vi "UHR-Fleezers Control (host) - 12.0(oscillate_test).vi"() -> ()   [LabVIEW 2014] (continued)
        n1224 = Divide(x=w1672, y="APD Integration Time (s)") -> (x/y=w1675:dbl)
        n1225 = Multiply(x=2.0, y=w1675) -> (x*y=w1674:dbl)
        n1226 = local write "APD Samples/FIFO Acq."(w1675) -> ()
        n1227 = local write "APD Elements/DMA read"(w1674) -> ()
      }
      event "Number of F/B Scans (AOD)", "Scan Speed (nm/s)", "Scan BD", "Initial D (MHz)", "Step Size (nm)", "Scan Range (nm)", "Wiggle amp 1 (units?)": Value Change {
        w1743 = 123.0  # AOM cal (nm/MHz)
        n1228 = event-data() -> ()  [unwired: 7 out]
        n1229 = local read "BD 1 Frequency 1 (MHz)"() -> (w1726:dbl)
        n1230 = local read "AOM X Cal (nm/MHz)"() -> (w1718:dbl)
        n1231 = local read "BD 2 Frequency 1 (MHz)"() -> (w1732:dbl)
        n1232 = local read "X RF Frequency Limits (MHz)"() -> (w1730:T17)
        n1233 = local read "Y RF Frequency Limits (MHz)"() -> (w1727:T17)
        n1234 = Negate(x="Scan Range (nm)") -> (-x=w1696:dbl)
        n1235 = Divide(x=w1696, y=w1718) -> (x/y=w1700:dbl)
        n1236 = Select(t=w1730, s="Scan BD", f=w1727) -> (s? t:f=w1729:T17)
        n1237 = Select(t=w1726, s="Scan BD", f=w1732) -> (s? t:f=w1731:dbl)
        n1238 = Unbundle By Name(w1729) -> ("Maximum"=w1738:dbl, "Minimum"=w1737:dbl)
        n1239 = Add(x=w1700, y=w1731) -> (x+y=w1735:dbl)
        n1240 = Divide(x=w1696, y="Step Size (nm)") -> (x/y=w1715:dbl)
        n1241 = Divide(x="Step Size (nm)", y=w1718) -> (x/y=w1724:dbl)
        n1242 = Absolute Value(x=w1715) -> (abs(x)=w1699:dbl)
        n1243 = Sign(1:w1696) -> (0:w1697:dbl)
        n1244 = In Range and Coerce(upper limit=w1738, x=w1735, lower limit=w1737) -> (coerced(x)=w1734:dbl, In Range?=w1736:bool)
        n1245 = To Unsigned Quad Integer(1:w1699) -> (0:w1714:u64)
        "Scan steps (AOD)" <- w1714
        n1246 = call "IR AOM freq to word.vi"("Frequency In (MHz)"=w1724) -> ("Frequency Word Out (double)"=w1721:dbl)
        n1247 = Multiply(x=w1697, y=w1721) -> (x*y=w1698:dbl)
        n1248 = Subtract(x=w1735, y=w1734) -> (x-y=w1733:dbl)
        n1249 = To Quad Integer(1:w1698) -> (0:w1720:i64)
        "Incr. int (AOD)" <- w1720
        n1250 = Subtract(x=w1700, y=w1733) -> (x-y=w1719:dbl)
        "Scan Range (MHz)" <- w1719
        n1251 = Select(t=w1700, s=w1736, f=w1719) -> (s? t:f=w1739:dbl)
        n1252 = Multiply(x=w1719, y=w1718) -> (x*y=w1717:dbl)
        n1253 = Decrement(x=w1714) -> (x-1=w1767:u64)
        n1254 = Negate(x=w1717) -> (-x=w1713:dbl)
        n1255 = local write "Scan Range (nm)"(w1713) -> ()
        n1256 = Divide(x=w1739, y=w1767) -> (x/y=w1723:dbl)
        "Scan Increment (MHz)" <- w1723
        n1257 = call "IR AOM freq to word.vi"("Frequency In (MHz)"=w1723) -> ("Frequency Word Out (double)"=w1722:dbl)
        n1258 = Divide(x="Step Size (nm)", y="Scan Speed (nm/s)") -> (x/y=w1710:dbl)
        n1259 = To Quad Integer(1:w1722) -> ()  [unwired: 1 out]
        n1260 = local read "Number Interlace Sets"() -> (w1694:u8)
        n1261 = local read "AI Count (ticks)"() -> (w1695:u32)
        n1262 = local read "Total Counts (ticks)"() -> (w1693:u32)
        n1263 = local read "# Samples/trap"() -> (w1725:u32)
        n1264 = Multiply(x=w1695, y=w1694) -> (x*y=w1692:u32)
        n1265 = Divide(x=w1693, y=w1692) -> (x/y=w1691:dbl)
        n1266 = Select(t=w1726, s="Scan BD", f=w1732) -> (s? t:f=w1764:dbl)
        "Initial freq. (MHz)" <- w1764
        n1267 = Add(x=w1739, y=w1764) -> (x+y=→"Final freq. (MHz)":dbl)
        n1268 = Divide(x=w1693, y=40000000.0) -> (x/y=w1709:dbl)
        n1269 = Divide(x=w1710, y=w1709) -> (x/y=w1708:dbl)
        n1270 = To Unsigned Quad Integer(1:w1708) -> (0:w1683:u64)
        n1271 = Quotient & Remainder(x=w1683, y=u64 2) -> (x-y*floor(x/y)=w1687:u64)  [unwired: 1 out]
        n1272 = Equal?(x=w1687, y=u64 0) -> (x = y?=w1685:bool)
        n1273 = Decrement(x=w1683) -> (x-1=w1684:u64)
        n1274 = Select(t=w1683, s=w1685, f=w1684) -> (s? t:f=w1682:u64)
        "Cycles/step (AOD)" <- w1682
        n1275 = xnode "Read/Write Control"("FPGA VI Reference In"=w1775, "error in"=w1774, "Scan steps"=w1714, "Number of scans"="Number of F/B Scans (AOD)", "Cycles per step"=w1682, "Scan freq.  increment"=w1720, "Scan BD"="Scan BD") -> ("error out"=w1773:errorcluster)  [unwired: 1 out]
        n1276 = Multiply(x=w1714, y=w1682) -> (x*y=w1768:u64)
        n1277 = Multiply(x=w1768, y=u64 2) -> (x*y=w1690:u64)
        n1278 = Multiply(x=w1691, y=w1690) -> (x*y=w1689:dbl)
        "Data points/scan (f/b)" <- w1689
        n1279 = Multiply(x=w1689, y="Number of F/B Scans (AOD)") -> (x*y=w1771:dbl)
        "Data points/scans" <- w1771
        n1280 = Divide(x=w1771, y=w1725) -> (x/y=→"N sets should be saved":dbl)
        n1281 = Multiply(x=w1768, y=w1709) -> (x*y=w1707:dbl)
        "Time/Scan (s) (AOD)" <- w1707
        n1282 = Select(t=w1739, s="Scan BD", f=0.0) -> (s? t:f=w1765:dbl)
        n1283 = Select(t=0.0, s="Scan BD", f=w1739) -> (s? t:f=w1761:dbl)
        n1284 = local read "BD 2 Frequency 2 (MHz)"() -> (w1757:dbl)
        n1285 = local read "BD 1 Frequency 2 (MHz)"() -> (w1760:dbl)
        n1286 = Add(x=w1761, y=w1732) -> (x+y=w1758:dbl)
        n1287 = Add(x=w1726, y=w1765) -> (x+y=w1759:dbl)
        n1288 = Multiply(x=w1707, y=2.0) -> (x*y=w1706:dbl)
        n1289 = Multiply(x=w1706, y="Number of F/B Scans (AOD)") -> (x*y=w1703:dbl)
        n1290 = Divide(x=w1703, y=60.0) -> (x/y=→"Time to Finish All (min)":dbl)
        n1291 = Add(x="Trap 2 Bead Size (nm)", y="Trap 1 Bead Size (nm)") -> (x+y=w1747:dbl)
        n1292 = Divide(x=w1747, y=2.0) -> (x/y=w1741:dbl)
        n1293 = Subtract(x=w1758, y=w1757) -> (x-y=w1755:dbl)
        n1294 = Subtract(x=w1759, y=w1760) -> (x-y=w1756:dbl)
        n1295 = local read "Initial D (MHz)"() -> (w1744:dbl)
        n1296 = Square(x=w1755) -> (x^2=w1754:dbl)
        n1297 = Square(x=w1756) -> (x^2=w1753:dbl)
        n1298 = Add(x=w1753, y=w1754) -> (x+y=w1752:dbl)
        n1299 = Square Root(x=w1752) -> (sqrt(x)=w1751:dbl)
        "Final D (MHz)" <- w1751
        n1300 = Multiply(x=w1743, y=w1751) -> (x*y=w1750:dbl)
        n1301 = Multiply(x=w1744, y=w1743) -> (x*y=w1742:dbl)
        n1302 = Subtract(x=w1742, y=w1741) -> (x-y=→"Initial sep (nm)":dbl)
        n1303 = Subtract(x=w1750, y=w1741) -> (x-y=→"Final sep (nm)":dbl)
      }
      event "Freq or Amp switch first", "Swap F1 and F2", "Freq switch delay", "Amp switch delay": Value Change {
        n1304 = event-data() -> ()  [unwired: 7 out]
        n1305 = local read "Freq or Amp switch first"() -> (w1776:bool)
        n1306 = local read "Amp switch delay"() -> (w1777:u16)
        n1307 = local read "Freq switch delay"() -> (w1779:u16)
        n1308 = local read "Swap F1 and F2"() -> (w1778:bool)
        n1309 = xnode "Read/Write Control"("FPGA VI Reference In"=w1782, "error in"=w1781, "Freq switch delay"=w1779, "Swap F1 and F2"=w1778, "Amp switch delay"=w1777, "Freq or Amp switch first"=w1776) -> ("error out"=w1780:errorcluster)  [unwired: 1 out]
      }
      event "Scan steps (MCL)", "Number of scans (MCL)", "Scan Range (V)\n(of steps)", "2D or 1D Scan", "N APD Samp/step", "Fast Scan Dir", "Continuous MCL Scanning", "Scan lines (y)": Value Change {
        w1784 = 32767.0 ("y")
        n1310 = event-data() -> ()  [unwired: 7 out]
        n1311 = Select(t="Scan lines (y)", s="2D or 1D Scan", f="Number of scans (MCL)") -> (s? t:f=w1789:u64)
        n1312 = Decrement(x="Scan steps (MCL)") -> (x-1=w1805:u64)
        n1313 = Divide(x="Scan Range (V)\n(of steps)", y=w1805) -> (x/y=w1804:dbl)
        "Desired Scan Incr (V)" <- w1804
        n1314 = local read "APD Integration Time (s)"() -> (w1797:dbl)
        n1315 = Multiply(x=w1804, y=w1784) -> (x*y=w1813:dbl)
        n1316 = Divide(x=w1813, y=10.0) -> (x/y=w1803:dbl)
        "Desired incr (int)" <- w1803
        n1317 = local read "Update Count (MCL)"() -> (w1809:u32)
        n1318 = Round Toward -Infinity(1:w1803) -> (0:w1812:dbl)
        n1319 = To Word Integer(number=w1812) -> (16bit integer=w1787:i16)
        "Actual Incr. int (MCL)" <- w1787
        n1320 = Multiply(x=w1797, y=40000000.0) -> (x*y=w1810:dbl)
        n1321 = Divide(x=w1810, y=w1809) -> (x/y=w1808:dbl)
        n1322 = Multiply(x=i16 10, y=w1787) -> (x*y=w1785:i16)
        n1323 = Multiply(x="N APD Samp/step", y=w1808) -> (x*y=w1807:dbl)
        "Cycles/step (MCL)" <- w1807
        n1324 = Divide(x=w1785, y=w1784) -> (x/y=→"Actual MCL Inc (V)":dbl)
        n1325 = Multiply(x="N APD Samp/step", y="Scan steps (MCL)") -> (x*y=w1799:dbl)
        n1326 = local read "APD Samples/FIFO Acq."() -> (w1796:dbl)
        n1327 = Multiply(x=w1799, y=u64 2) -> (x*y=w1798:dbl)
        "Data points/scan (f+b)" <- w1798
        n1328 = Multiply(x=w1798, y=w1789) -> (x*y=w1816:dbl)
        "Data points/scans (MCL)" <- w1816
        n1329 = Multiply(x=w1797, y=w1798) -> (x*y=w1790:dbl)
        "Time/f+b scan (s) (MCL)" <- w1790
        n1330 = Divide(x=w1816, y=w1796) -> (x/y=→"N sets should be saved (MCL)":dbl)
        n1331 = Multiply(x=w1790, y=w1789) -> (x*y=→"Total Time (s)":dbl)
        n1332 = Not(x="Fast Scan Dir") -> (.not. x?=w1794:bool)
        n1333 = xnode "Read/Write Control"("FPGA VI Reference In"=w1820, "error in"=w1819, "Scan steps (MCL)"="Scan steps (MCL)", "Number of scans (MCL)"=w1789, "Cycles per step (MCL)"=w1807, "Scan freq.  increment (MCL)"=w1787, "1D or 2D Scan?"="2D or 1D Scan", "MCL Scan Axis"=w1794, "Cont. Scan (MCL)"="Continuous MCL Scanning") -> ("error out"=w1818:errorcluster)  [unwired: 1 out]
      }
      event "Read Cal": Value Change {
        w1822 = 1000.0 ("y")
        n1334 = event-data() -> ()  [unwired: 7 out]
        n1335 = local read "Save file name"() -> (w1847:path)
        n1336 = local write "Read Cal"(FALSE ("Read Cal")) -> ()
        n1337 = Strip Path(path=w1847) -> (stripped path=w1846:path)  [unwired: 1 out]
        n1338 = Path To String(path=w1846) -> (string=w1845:string)
        n1339 = Concatenate Strings(w1845, "\\current.cal" ("string")) -> (w1843:string)
        n1340 = String To Path(string=w1843) -> (path=w1842:path)
        n1341 = Open/Create/Replace File(file path (use dialog)=w1842, operation (0:open)=T30."open", access (0:read/write)=enum16{"read/write", "read-only", "write-only"}."read-only") -> (refnum out=w1850:refnum<file>, error out=w1836:errorcluster)  [unwired: 1 in, 3 out]
        n1342 = Deny Access(4:w1836, 7:w1850) -> (0:w1835:errorcluster, 3:w1841:refnum<file>)  [unwired: 1 out]
        n1343 = Read from Binary File(5:0.0, 8:w1835, 9:T29."big-endian, network order" ("byte order (0:big-endian, network order)"), 10:-1 ("count (1)"), 11:w1841) -> (0:w1834:errorcluster, 2:w1832:dbl[], 3:w1837:refnum<file>)  [unwired: 2 out]
        n1344 = Array To Cluster(array=w1832) -> (cluster=w1831:T32)
        n1345 = Unbundle(w1831) -> ("[0]"=w1830:dbl, "[1]"=w1829:dbl, "[2]"=w1828:dbl, "[3]"=w1827:dbl, "[4]"=w1826:dbl, "[5]"=w1825:dbl)
        n1346 = Close File(refnum=w1837, error in=w1834) -> (error out=→"Read cal error":errorcluster)  [unwired: 1 out]
        n1347 = Multiply(x=w1825, y=w1822) -> (x*y=w1823:dbl)
        n1348 = local write "T2 k_x (pN/nm)"(w1827) -> ()
        n1349 = local write "T1 k_x (pN/nm)"(w1828) -> ()
        n1350 = local write "T1 a_x (nm/V)"(w1830) -> ()
        n1351 = local write "T2 a_x (nm/V)"(w1829) -> ()
        n1352 = Multiply(x=w1826, y=w1822) -> (x*y=w1824:dbl)
        n1353 = local write "T1 offset_x (mV)"(w1824) -> ()
        n1354 = local write "T2 offset_x (mV)"(w1823) -> ()
      }
      event "Read FX file": Value Change {
        n1355 = event-data() -> ()  [unwired: 7 out]
        n1356 = local write "Read FX file"(FALSE ("Read residual")) -> ()
        n1357 = local read "Save file name"() -> (w1875:path)
        n1358 = Strip Path(path=w1875) -> (stripped path=w1874:path)  [unwired: 1 out]
        n1359 = Path To String(path=w1874) -> (string=w1873:string)
        n1360 = Concatenate Strings(w1873, "\\current.cal" ("string")) -> (w1871:string)
        n1361 = String To Path(string=w1871) -> (path=w1870:path)
        n1362 = Open/Create/Replace File(file path (use dialog)=w1870, operation (0:open)=T30."open", access (0:read/write)=enum16{"read/write", "read-only", "write-only"}."read-only") -> (refnum out=w1867:refnum<file>, error out=w1864:errorcluster)  [unwired: 3 in, 1 out]
        n1363 = Deny Access(4:w1864, 7:w1867) -> (0:w1863:errorcluster, 3:w1866:refnum<file>)  [unwired: 1 in]
        n1364 = Read from Binary File(5:0.0, 8:w1863, 9:T29."big-endian, network order" ("byte order (0:big-endian, network order)"), 10:-1 ("count"), 11:w1866) -> (0:w1859:errorcluster, 2:w1853:dbl[], 3:w1860:refnum<file>)  [unwired: 1 in, 1 out]
        n1365 = Index Array(array=w1853, index=6) -> (element=→"Bad fit error":dbl)
        n1366 = Index Array(array=w1853, index=7) -> (element=→"Fit offset":dbl)
        n1367 = Index Array(array=w1853, index=8) -> (element=→"Hyst. error":dbl)
        n1368 = Close File(refnum=w1860, error in=w1859) -> ()  [unwired: 2 out]
      }
      event "Abort MCL Scan": Value Change {
        n1369 = event-data() -> ()  [unwired: 7 out]
        n1370 = local write "MCL Scanning"(FALSE ("MCL Scanning")) -> ()
        n1371 = xnode "Read/Write Control"("FPGA VI Reference In"=w1880, "error in"=w1879, "Abort scan (MCL)"="Abort MCL Scan") -> ("error out"=w1878:errorcluster)  [unwired: 1 out]
      }
      event "Update Count (MCL)": Value Change {
        n1372 = event-data() -> ()  [unwired: 7 out]
        n1373 = xnode "Read/Write Control"("FPGA VI Reference In"=w1884, "error in"=w1883, "MCL count"="Update Count (MCL)") -> ("error out"=w1882:errorcluster)  [unwired: 1 out]
      }
      event "Phase adjust (MCL)", "+ phase (MCL)", "- phase (MCL)": Value Change {
        n1374 = event-data() -> ()  [unwired: 7 out]
        n1375 = Negate(x="Phase adjust (MCL)") -> (-x=w1893:i16)
        n1376 = Select(t=w1893, s="- phase (MCL)", f="Phase adjust (MCL)") -> (s? t:f=w1891:i16)
        n1377 = Or(x="- phase (MCL)", y="+ phase (MCL)") -> (x .or. y?=w1886:bool)
        n1378 = xnode "Read/Write Control"("FPGA VI Reference In"=w1895, "error in"=w1894, "Phase count adjustment (MCL)"=w1891) -> ("FPGA VI Reference Out"=w1887:T22, "error out"=w1888:errorcluster)
        n1379 = xnode "Read/Write Control"("FPGA VI Reference In"=w1887, "error in"=w1888, "+ phase (MCL)"=w1886) -> ("error out"=w1885:errorcluster)  [unwired: 1 out]
      }
      event "Abort AOD Scan": Value Change {
        n1380 = event-data() -> ()  [unwired: 7 out]
        n1381 = xnode "Read/Write Control"("FPGA VI Reference In"=w1899, "error in"=w1898, "Abort scan"="Abort AOD Scan") -> ("error out"=w1897:errorcluster)  [unwired: 1 out]
      }
      event "Continuous AOD Scanning": Value Change {
        n1382 = event-data() -> ()  [unwired: 7 out]
        n1383 = xnode "Read/Write Control"("FPGA VI Reference In"=w1903, "error in"=w1902, "Cont. Scan"="Continuous AOD Scanning") -> ("error out"=w1901:errorcluster)  [unwired: 1 out]
      }
      event "Index": Value Change {
        n1384 = event-data() -> ()  [unwired: 7 out]
        n1385 = call "Create new save file.vi"("Insert"="", "Ext"=".dat" ("string"), "Index In"="Index") -> ("Path Out"=→"Save file name":path, "Index Out"=w1904:dbl)
        "Save index" <- w1904
        n1386 = local write "Index"(w1904) -> ()
      }
      event "AO1", "AO2": Value Change {
        w1919 = 10.0 ("y")
        w1918 = 32767.0 ("y")
        n1387 = event-data() -> ()  [unwired: 7 out]
        n1388 = local read "AO2"() -> (w1917:dbl)
        n1389 = local read "AO1"() -> (w1914:dbl)
        n1390 = Multiply(x=w1914, y=w1918) -> (x*y=w1913:dbl)
        n1391 = Multiply(x=w1917, y=w1918) -> (x*y=w1916:dbl)
        n1392 = Divide(x=w1913, y=w1919) -> (x/y=w1912:dbl)
        n1393 = Divide(x=w1916, y=w1919) -> (x/y=w1915:dbl)
        n1394 = To Word Integer(number=w1912) -> (16bit integer=w1920:i16)
        n1395 = To Word Integer(number=w1915) -> (16bit integer=w1921:i16)
        n1396 = xnode "Read/Write Control"("FPGA VI Reference In"=w1911, "error in"=w1910, "AO1"=w1920, "AO2"=w1921) -> ("error out"=w1909:errorcluster)  [unwired: 1 out]
      }
      event "Inject Pump 1": Value Change {
        n1397 = event-data() -> ()  [unwired: 7 out]
        n1398 = local read "Use Harvard pumps\nfor beads (else Chemyx)"() -> (w1923:bool)
        n1399 = case shown="True" w1923 {
          tunnel: "Inject Pump 1" -> [w1927 w1965]
          tunnel: w1922 -> [_ w1966]
          frame False {
            n1400 = local read "Pump write delay (ms)"() -> (w1926:dbl)
            n1401 = local read "Chemyx Syringe Pump Serial Port"() -> (w1925:refnum<visa-resource-name>)
            n1402 = case shown="True" w1927 {
              tunnel: w1926 -> [w1933 w1947]
              tunnel: w1925 -> [w1930 w1946]
              frame False {
                n1403 = flat-sequence {
                  tunnel: w1930 -> [w1934]
                  tunnel: [w1934] -> w1931
                  tunnel: w1933 -> [_]
                  tunnel: [w1937] -> w1932
                  tunnel: w1931 -> [w1937]
                  tunnel: w1932 -> [w1938]
                  tunnel: [w1938] -> w1928
                  tunnel: [w1940] -> w1929
                  tunnel: w1928 -> [w1940]
                  tunnel: w1929 -> [w1942]
                  frame #0 {
                    n1404 = call "Write to pump.vi"("string"="enter pump1", "VISA resource name"=w1934) -> ()  [unwired: 1 out]
                  }
                  frame #1 {
                    n1405 = Wait (ms)(milliseconds to wait="Pump pause delay (ms)") -> ()  [unwired: 1 out]
                  }
                  frame #2 {
                    n1406 = call "Write to pump.vi"("string"="stop", "VISA resource name"=w1938) -> ()  [unwired: 1 out]
                  }
                  frame #3 {
                    n1407 = Wait (ms)(milliseconds to wait=u32 500) -> ()  [unwired: 1 out]
                  }
                  frame #4 {
                    n1408 = call "Write to pump.vi"("string"="stop", "VISA resource name"=w1942) -> ()  [unwired: 1 out]
                  }
                }
              }
              frame True {
                n1409 = flat-sequence {
                  tunnel: w1946 -> [w1956]
                  tunnel: w1947 -> [w1951]
                  tunnel: w1947 -> [w1958]
                  tunnel: w1946 -> [w1959]
                  tunnel: [w1959] -> w1944
                  tunnel: [w1961] -> w1945
                  tunnel: w1944 -> [w1961]
                  tunnel: w1945 -> [w1963]
                  frame #0 {
                    n1410 = local read "All Pump Parameters"() -> (w1950:T5)
                    n1411 = Unbundle By Name(w1950) -> ("Pump 1"=w1957:T33)
                    n1412 = call "Set pump parameters.vi"("Pump write delay (ms)"=w1951, "Volume (uL)"="Ch 1 Inject Volume (uL)", "Rate (uL/h)"="Ch 1 Inject Rate (ul/h)", "Units"=4.0, "Pump #"=1.0, "Pump Parameters In"=w1957, "VISA resource name"=w1956) -> ("Pump Parameters Out"=w1949:T33)  [unwired: 3 in]
                    n1413 = Bundle By Name(cluster=w1950, "Pump 1"=w1949) -> (w1948:T5)
                    n1414 = local write "All Pump Parameters"(w1948) -> ()
                  }
                  frame #1 {
                    n1415 = Wait (ms)(milliseconds to wait=w1958) -> ()  [unwired: 1 out]
                  }
                  frame #2 {
                    n1416 = call "Write to pump.vi"("string"="start", "VISA resource name"=w1959) -> ()  [unwired: 1 out]
                  }
                  frame #3 {
                    n1417 = Wait (ms)(milliseconds to wait=u32 500) -> ()  [unwired: 1 out]
                  }
                  frame #4 {
                    n1418 = call "Write to pump.vi"("string"="start", "VISA resource name"=w1963) -> ()  [unwired: 1 out]
                  }
                }
              }
            }
          }
          frame True {
            n1419 = case shown="True" w1965 {
              tunnel: w1966 -> [w1967 w1977]
              frame False {
                n1420 = flat-sequence {
                  tunnel: w1967 -> [w1969]
                  frame #0 {
                    n1421 = local write "Flushing P1"(FALSE ("Flushing P1")) -> ()
                    n1422 = Concatenate Strings("stop" ("string"), "\r") -> (w1971:string)
                    n1423 = VISA Write(VISA resource name=w1969, write buffer=w1971) -> ()  [unwired: 1 in, 3 out]
                  }
                  frame #1 {
                    n1424 = property on="Clear Volume P1" class="Bool (strict)"("Val(Sgnl)"=TRUE ("Value (Signaling)")) -> ()  [unwired: 2 in, 2 out]
                  }
                }
              }
              frame True {
                n1425 = local read "Normal Flow Rate (ul/h) P1"() -> (w1975:dbl)
                n1426 = Number To Decimal String(number=w1975) -> (decimal integer string=w1981:string)  [unwired: 1 in]
                n1427 = Concatenate Strings("irate  " ("string"), w1981, " u/h" ("string"), "\r") -> (w1979:string)
                n1428 = VISA Write(VISA resource name=w1977, write buffer=w1979) -> (VISA resource name out=w1976:refnum<visa-resource-name>)  [unwired: 1 in, 2 out]
                n1429 = Concatenate Strings("irun" ("string"), "\r") -> (w1983:string)
                n1430 = VISA Write(VISA resource name=w1976, write buffer=w1983) -> ()  [unwired: 1 in, 3 out]
              }
            }
          }
        }
      }
      event "Inject Pump 3": Value Change {
        n1431 = event-data() -> ()  [unwired: 7 out]
        n1432 = local read "Use Harvard pumps\nfor beads (else Chemyx)"() -> (w1986:bool)
        n1433 = case shown="True" w1986 {
          tunnel: "Inject Pump 3" -> [w1990 w2029]
          tunnel: w1985 -> [_ w2028]
          frame False {
            n1434 = local read "Pump write delay (ms)"() -> (w1989:dbl)
            n1435 = case shown="True" w1990 {
              tunnel: w1989 -> [w1996 w2010]
              tunnel: "Chemyx Syringe Pump Serial Port" -> [w1993 w2009]
              frame False {
                n1436 = flat-sequence {
                  tunnel: w1993 -> [w1997]
                  tunnel: [w1997] -> w1994
                  tunnel: w1996 -> [_]
                  tunnel: [w2000] -> w1995
                  tunnel: w1994 -> [w2000]
                  tunnel: w1995 -> [w2001]
                  tunnel: [w2001] -> w1991
                  tunnel: [w2003] -> w1992
                  tunnel: w1991 -> [w2003]
                  tunnel: w1992 -> [w2005]
                  frame #0 {
                    n1437 = call "Write to pump.vi"("string"="enter pump3", "VISA resource name"=w1997) -> ()  [unwired: 1 out]
                  }
                  frame #1 {
                    n1438 = local read "Pump pause delay (ms)"() -> (w1999:u32)
                    n1439 = Wait (ms)(milliseconds to wait=w1999) -> ()  [unwired: 1 out]
                  }
                  frame #2 {
                    n1440 = call "Write to pump.vi"("string"="stop", "VISA resource name"=w2001) -> ()  [unwired: 1 out]
                  }
                  frame #3 {
                    n1441 = Wait (ms)(milliseconds to wait=u32 0) -> ()  [unwired: 1 out]
                  }
                  frame #4 {
                    n1442 = call "Write to pump.vi"("string"="stop", "VISA resource name"=w2005) -> ()  [unwired: 1 out]
                  }
                }
              }
              frame True {
                n1443 = flat-sequence {
                  tunnel: w2009 -> [w2019]
                  tunnel: w2010 -> [w2014]
                  tunnel: w2010 -> [w2021]
                  tunnel: w2009 -> [w2022]
                  tunnel: [w2022] -> w2008
                  tunnel: [w2025] -> w2007
                  tunnel: w2008 -> [w2025]
                  tunnel: w2007 -> [w2026]
                  frame #0 {
                    n1444 = local read "All Pump Parameters"() -> (w2013:T5)
                    n1445 = Unbundle By Name(w2013) -> ("Pump 3"=w2020:T33)
                    n1446 = call "Set pump parameters.vi"("Pump write delay (ms)"=w2014, "Volume (uL)"="Ch 3 Inject Volume (uL)", "Rate (uL/h)"="Ch 3 Inject Rate (ul/h)", "Units"=4.0, "Pump #"=3.0, "Pump Parameters In"=w2020, "VISA resource name"=w2019) -> ("Pump Parameters Out"=w2012:T33)  [unwired: 3 in]
                    n1447 = Bundle By Name(cluster=w2013, "Pump 3"=w2012) -> (w2011:T5)
                    n1448 = local write "All Pump Parameters"(w2011) -> ()
                  }
                  frame #1 {
                    n1449 = Wait (ms)(milliseconds to wait=w2021) -> ()  [unwired: 1 out]
                  }
                  frame #2 {
                    n1450 = call "Write to pump.vi"("string"="start", "VISA resource name"=w2022) -> ()  [unwired: 1 out]
                  }
                  frame #3 {
                    n1451 = Wait (ms)(milliseconds to wait=u32 500) -> ()  [unwired: 1 out]
                  }
                  frame #4 {
                    n1452 = call "Write to pump.vi"("string"="start", "VISA resource name"=w2026) -> ()  [unwired: 1 out]
                  }
                }
              }
            }
          }
          frame True {
            n1453 = case shown="True" w2029 {
              tunnel: w2028 -> [w2030 w2037]
              frame False {
                n1454 = flat-sequence {
                  tunnel: w2030 -> [w2032]
                  frame #0 {
                    n1455 = local write "Flushing P3"(FALSE ("Flushing P3")) -> ()
                    n1456 = Concatenate Strings("stop" ("string"), "\r") -> (w2034:string)
                    n1457 = VISA Write(VISA resource name=w2032, write buffer=w2034) -> ()  [unwired: 1 in, 3 out]
                  }
                  frame #1 {
                    n1458 = property on="Clear Volume P3" class="Bool (strict)"("Val(Sgnl)"=TRUE ("Value (Signaling)")) -> ()  [unwired: 2 in, 2 out]
                  }
                }
              }
              frame True {
                n1459 = local read "Normal Flow Rate (ul/h) P3"() -> (w2038:dbl)
                n1460 = Number To Decimal String(number=w2038) -> (decimal integer string=w2044:string)  [unwired: 1 in]
                n1461 = Concatenate Strings("irate  " ("string"), w2044, " u/h" ("string"), "\r") -> (w2042:string)
                n1462 = VISA Write(VISA resource name=w2037, write buffer=w2042) -> (VISA resource name out=w2040:refnum<visa-resource-name>)  [unwired: 1 in, 2 out]
                n1463 = Concatenate Strings("irun" ("string"), "\r") -> (w2046:string)
                n1464 = VISA Write(VISA resource name=w2040, write buffer=w2046) -> ()  [unwired: 1 in, 3 out]
              }
            }
          }
        }
      }
      event "Inject Pump 2": Value Change {
        n1465 = event-data() -> ()  [unwired: 7 out]
        n1466 = local read "Pump write delay (ms)"() -> (w2050:dbl)
        n1467 = local read "Chemyx Syringe Pump Serial Port"() -> (w2048:refnum<visa-resource-name>)
        n1468 = flat-sequence {
          tunnel: w2048 -> [w2063]
          tunnel: w2050 -> [w2059]
          tunnel: "Inject Pump 2" -> [_]
          tunnel: w2050 -> [w2065]
          tunnel: w2048 -> [w2066]
          frame #0 {
            n1469 = local read "All Pump Parameters"() -> (w2058:T5)
            n1470 = Multiply(x=60.0, y="Flush Center Ch Rate (ul/m)") -> (x*y=w2055:dbl)
            n1471 = Unbundle By Name(w2058) -> ("Pump 2"=w2064:T33)
            n1472 = call "Set pump parameters.vi"("Pump write delay (ms)"=w2059, "Volume (uL)"="Flush Center Ch Volume (uL)", "Rate (uL/h)"=w2055, "Units"=3.0, "Pump #"=2.0, "Pump Parameters In"=w2064, "VISA resource name"=w2063) -> ("Pump Parameters Out"=w2057:T33)  [unwired: 3 in]
            n1473 = Bundle By Name(cluster=w2058, "Pump 2"=w2057) -> (w2056:T5)
            n1474 = Add(x="Flush Center Ch Volume (uL)", y="Total Volume\nFlushed (uL)") -> (x+y=w2052:dbl)
            n1475 = local write "All Pump Parameters"(w2056) -> ()
            n1476 = local write "Total Volume\nFlushed (uL)"(w2052) -> ()
          }
          frame #1 {
            n1477 = Wait (ms)(milliseconds to wait=w2065) -> ()  [unwired: 1 out]
          }
          frame #2 {
            n1478 = call "Write to pump.vi"("string"="start", "VISA resource name"=w2066) -> ()  [unwired: 1 out]
          }
        }
      }
      event "Sample Channel\nFlow": Value Change {
        n1479 = event-data() -> ()  [unwired: 7 out]
        n1480 = case shown="True" "Sample Channel\nFlow" {
          tunnel: w2069 -> [w2070 w2076]
          frame False {
            n1481 = flat-sequence {
              tunnel: w2070 -> [w2072]
              frame #0 {
                n1482 = local write "Flushing samp"(FALSE ("Flushing samp")) -> ()
                n1483 = Concatenate Strings("stop" ("string"), "\r") -> (w2075:string)
                n1484 = VISA Write(VISA resource name=w2072, write buffer=w2075) -> ()  [unwired: 1 in, 3 out]
              }
            }
          }
          frame True {
            n1485 = local read "Normal Flow rate (mL/h)"() -> (w2086:dbl)
            n1486 = Number To Decimal String(number=w2086) -> (decimal integer string=w2085:string)  [unwired: 1 in]
            n1487 = Concatenate Strings("irate " ("string"), w2085, " u/h" ("string"), "\r") -> (w2081:string)
            n1488 = VISA Write(VISA resource name=w2076, write buffer=w2081) -> (VISA resource name out=w2080:refnum<visa-resource-name>)  [unwired: 1 in, 2 out]
            n1489 = Concatenate Strings("irun" ("string"), "\r") -> (w2077:string)
            n1490 = VISA Write(VISA resource name=w2080, write buffer=w2077) -> ()  [unwired: 1 in, 3 out]
          }
        }
      }
      event "Start Flow": Value Change {
        n1491 = event-data() -> ()  [unwired: 7 out]
        n1492 = local write "Sample Channel\nFlow"(TRUE ("Sample Channel\nFlow")) -> ()
        n1493 = local write "Start Flow"(FALSE ("Start Flow")) -> ()
        n1494 = Concatenate Strings("irun" ("string"), "\r") -> (w2091:string)
        n1495 = VISA Write(VISA resource name=w2087, write buffer=w2091) -> ()  [unwired: 1 in, 3 out]
      }
      event "Stop Flow": Value Change {
        w2093 = FALSE ("Stop Flow")
        n1496 = event-data() -> ()  [unwired: 7 out]
        n1497 = local write "Stop Flow"(w2093) -> ()
        n1498 = local write "Sample Channel\nFlow"(w2093) -> ()
        n1499 = Concatenate Strings("stop" ("string"), "\r") -> (w2096:string)
        n1500 = VISA Write(VISA resource name=w2094, write buffer=w2096) -> ()  [unwired: 1 in, 3 out]
      }
      event "Normal Flow rate (mL/h)": Value Change {
        n1501 = event-data() -> ()  [unwired: 7 out]
        n1502 = Number To Decimal String(number="Normal Flow rate (mL/h)") -> (decimal integer string=w2103:string)  [unwired: 1 in]
        n1503 = Concatenate Strings("irate  " ("string"), w2103, " u/h" ("string"), "\r") -> (w2102:string)
        n1504 = VISA Write(VISA resource name=w2099, write buffer=w2102) -> ()  [unwired: 1 in, 3 out]
      }
      event "Flush Sample": Value Change {
        n1505 = event-data() -> ()  [unwired: 7 out]
        n1506 = flat-sequence {
          tunnel: w2105 -> [w2133]
          frame #0 {
            # "set parameters (rate, volume) for flush, clear volume"
            n1507 = Number To Decimal String(number="Flush rate (mL/m)") -> (decimal integer string=w2129:string)  [unwired: 1 in]
            n1508 = local write "Sample Channel\nFlow"(TRUE ("Sample Channel\nFlow")) -> ()
            n1509 = Concatenate Strings("irate  " ("string"), w2129, " u/m" ("string"), "\r") -> (w2131:string)
            n1510 = VISA Write(VISA resource name=w2133, write buffer=w2131) -> (VISA resource name out=w2127:refnum<visa-resource-name>)  [unwired: 1 in, 2 out]
            n1511 = Number To Decimal String(number="Flush volume (mL)") -> (decimal integer string=w2118:string)  [unwired: 1 in]
            n1512 = Reciprocal(x="Flush rate (mL/m)") -> (1/x=w2112:dbl)
            n1513 = Concatenate Strings("tvolume  " ("string"), w2118, " u" ("string"), "\r") -> (w2116:string)
            n1514 = Multiply(x=w2112, y="Flush volume (mL)") -> (x*y=w2110:dbl)
            n1515 = VISA Write(VISA resource name=w2127, write buffer=w2116) -> (VISA resource name out=w2115:refnum<visa-resource-name>)  [unwired: 1 in, 2 out]
            n1516 = Multiply(x=w2110, y=60.0) -> (x*y=→"Samp Flush Time (s)":dbl)
            n1517 = Concatenate Strings("cvolume" ("string"), "\r") -> (w2114:string)
            n1518 = VISA Write(VISA resource name=w2115, write buffer=w2114) -> (VISA resource name out=w2125:refnum<visa-resource-name>)  [unwired: 1 in, 2 out]
            n1519 = Concatenate Strings("irun" ("string"), "\r") -> (w2123:string)
            n1520 = VISA Write(VISA resource name=w2125, write buffer=w2123) -> ()  [unwired: 1 in, 3 out]
          }
          frame #1 {
            "Flushing samp" <- TRUE ("Boolean")
          }
        }
      }
      event "Flush Pump 3": Value Change {
        n1521 = event-data() -> ()  [unwired: 7 out]
        n1522 = flat-sequence {
          tunnel: w2135 -> [w2138]
          frame #0 {
            # "set paramaters (rate, volume) for flush, clear volume"
            n1523 = Number To Decimal String(number="Flush rate (uL/m) P3") -> (decimal integer string=w2160:string)  [unwired: 1 in]
            n1524 = local write "Inject Pump 3"(TRUE ("Inject Pump 3")) -> ()
            n1525 = Concatenate Strings("irate  " ("string"), w2160, " u/m" ("string"), "\r") -> (w2162:string)
            n1526 = VISA Write(VISA resource name=w2138, write buffer=w2162) -> (VISA resource name out=w2158:refnum<visa-resource-name>)  [unwired: 1 in, 2 out]
            n1527 = Reciprocal(x="Flush rate (uL/m) P3") -> (1/x=w2142:dbl)
            n1528 = Number To Decimal String(number="Volume (uL) P3") -> (decimal integer string=w2149:string)  [unwired: 1 in]
            n1529 = Multiply(x="Volume (uL) P3", y=w2142) -> (x*y=w2141:dbl)
            n1530 = Concatenate Strings("tvolume  " ("string"), w2149, " u" ("string"), "\r") -> (w2147:string)
            n1531 = Multiply(x=w2141, y=60.0) -> (x*y=→"HP3 Flush Time (s)":dbl)
            n1532 = VISA Write(VISA resource name=w2158, write buffer=w2147) -> (VISA resource name out=w2146:refnum<visa-resource-name>)  [unwired: 1 in, 2 out]
            n1533 = Concatenate Strings("cvolume" ("string"), "\r") -> (w2145:string)
            n1534 = VISA Write(VISA resource name=w2146, write buffer=w2145) -> (VISA resource name out=w2156:refnum<visa-resource-name>)  [unwired: 1 in, 2 out]
            n1535 = Concatenate Strings("irun" ("string"), "\r") -> (w2154:string)
            n1536 = VISA Write(VISA resource name=w2156, write buffer=w2154) -> ()  [unwired: 1 in, 3 out]
          }
          frame #1 {
            "Flushing P3" <- TRUE ("Flushing P3")
          }
        }
      }
      event "Flush Pump 1": Value Change {
        n1537 = event-data() -> ()  [unwired: 7 out]
        n1538 = flat-sequence {
          tunnel: [w2176] -> w2166
          tunnel: w2165 -> [w2169]
          tunnel: w2166 -> [_]
          frame #0 {
            # "set paramaters (rate, volume) for flush, clear volume"
            n1539 = local write "Inject Pump 1"(TRUE ("Inject Pump 1")) -> ()
            n1540 = Number To Decimal String(number="Flush rate (uL/m) P1") -> (decimal integer string=w2192:string)  [unwired: 1 in]
            n1541 = Concatenate Strings("irate  " ("string"), w2192, " u/m" ("string"), "\r") -> (w2194:string)
            n1542 = VISA Write(VISA resource name=w2169, write buffer=w2194) -> (VISA resource name out=w2190:refnum<visa-resource-name>)  [unwired: 1 in, 2 out]
            n1543 = Reciprocal(x="Flush rate (uL/m) P1") -> (1/x=w2173:dbl)
            n1544 = Number To Decimal String(number="Volume (uL) P1") -> (decimal integer string=w2181:string)  [unwired: 1 in]
            n1545 = Multiply(x="Volume (uL) P1", y=w2173) -> (x*y=w2172:dbl)
            n1546 = Concatenate Strings("tvolume  " ("string"), w2181, " u" ("string"), "\r") -> (w2179:string)
            n1547 = Multiply(x=w2172, y=60.0) -> (x*y=→"HP1 Flush Time (s)":dbl)
            n1548 = VISA Write(VISA resource name=w2190, write buffer=w2179) -> (VISA resource name out=w2178:refnum<visa-resource-name>)  [unwired: 1 in, 2 out]
            n1549 = Concatenate Strings("cvolume" ("string"), "\r") -> (w2177:string)
            n1550 = VISA Write(VISA resource name=w2178, write buffer=w2177) -> (VISA resource name out=w2188:refnum<visa-resource-name>)  [unwired: 1 in, 2 out]
            n1551 = Concatenate Strings("irun" ("string"), "\r") -> (w2186:string)
            n1552 = VISA Write(VISA resource name=w2188, write buffer=w2186) -> (VISA resource name out=w2176:refnum<visa-resource-name>)  [unwired: 1 in, 2 out]
          }
          frame #1 {
            "Flushing P1" <- TRUE ("Flushing P3")
          }
        }
      }
      event "Clear Volume": Value Change {
        n1553 = event-data() -> ()  [unwired: 7 out]
        n1554 = Number To Decimal String(number="Normal volume (mL)") -> (decimal integer string=w2201:string)  [unwired: 1 in]
        n1555 = Concatenate Strings("tvolume " ("string"), w2201, " u" ("string"), "\r") -> (w2198:string)
        n1556 = VISA Write(VISA resource name=w2204, write buffer=w2198) -> (VISA resource name out=w2197:refnum<visa-resource-name>)  [unwired: 1 in, 2 out]
        n1557 = local write "Clear Volume"(FALSE ("Clear Volume")) -> ()
        n1558 = Concatenate Strings("cvolume" ("string"), "\r") -> (w2206:string)
        n1559 = VISA Write(VISA resource name=w2197, write buffer=w2206) -> ()  [unwired: 1 in, 3 out]
      }
      event "Clear Volume P3": Value Change {
        n1560 = event-data() -> ()  [unwired: 7 out]
        n1561 = Concatenate Strings("cvolume" ("string"), "\r") -> (w2212:string)
        n1562 = VISA Write(VISA resource name=w2211, write buffer=w2212) -> ()  [unwired: 1 in, 3 out]
        n1563 = local write "Clear Volume P3"(FALSE ("Clear Volume P3")) -> ()
      }
      event "Clear Volume P1": Value Change {
        n1564 = event-data() -> ()  [unwired: 7 out]
        n1565 = Concatenate Strings("cvolume" ("string"), "\r") -> (w2217:string)
        n1566 = local write "Clear Volume P1"(FALSE ("Clear Volume P1")) -> ()
        n1567 = VISA Write(VISA resource name=w2216, write buffer=w2217) -> ()  [unwired: 1 in, 3 out]
      }
      event "Display On P3": Value Change {
        n1568 = event-data() -> ()  [unwired: 7 out]
        n1569 = Select(t="dim 100", s="Display On P3", f="dim 0") -> (s? t:f=w2223:string)
        n1570 = Concatenate Strings(w2223, "\r") -> (w2225:string)
        n1571 = VISA Write(VISA resource name=w2220, write buffer=w2225) -> ()  [unwired: 1 in, 3 out]
      }
      event "Display On P1": Value Change {
        n1572 = event-data() -> ()  [unwired: 7 out]
        n1573 = Select(t="dim 100", s="Display On P1", f="dim 0") -> (s? t:f=w2230:string)
        n1574 = Concatenate Strings(w2230, "\r") -> (w2232:string)
        n1575 = VISA Write(VISA resource name=w2227, write buffer=w2232) -> ()  [unwired: 1 in, 3 out]
      }
      event "Retract Pump 3": Value Change {
        n1576 = event-data() -> ()  [unwired: 7 out]
        n1577 = local write "Retract Pump 3"(FALSE ("Retract Pump 3")) -> ()
        n1578 = case shown="True" "Retract Pump 3" {
          tunnel: w2234 -> [_ w2237]
          frame False {
          }
          frame True {
            n1579 = Number To Decimal String(number="Retract Rate (mL/m)") -> (decimal integer string=w2255:string)  [unwired: 1 in]
            n1580 = Concatenate Strings("wrate  " ("string"), w2255, " u/m" ("string"), "\r") -> (w2257:string)
            n1581 = VISA Write(VISA resource name=w2237, write buffer=w2257) -> (VISA resource name out=w2248:refnum<visa-resource-name>)  [unwired: 1 in, 2 out]
            n1582 = Number To Decimal String(number="Retract Vol 3 (uL)") -> (decimal integer string=w2250:string)  [unwired: 1 in]
            n1583 = Concatenate Strings("tvolume  " ("string"), w2250, " u" ("string"), "\r") -> (w2247:string)
            n1584 = VISA Write(VISA resource name=w2248, write buffer=w2247) -> (VISA resource name out=w2243:refnum<visa-resource-name>)  [unwired: 1 in, 2 out]
            n1585 = Concatenate Strings("cvolume" ("string"), "\r") -> (w2244:string)
            n1586 = VISA Write(VISA resource name=w2243, write buffer=w2244) -> (VISA resource name out=w2238:refnum<visa-resource-name>)  [unwired: 1 in, 2 out]
            n1587 = Concatenate Strings("wrun" ("string"), "\r") -> (w2239:string)
            n1588 = VISA Write(VISA resource name=w2238, write buffer=w2239) -> ()  [unwired: 1 in, 3 out]
          }
        }
      }
      event "Retract Pump 1": Value Change {
        n1589 = event-data() -> ()  [unwired: 7 out]
        n1590 = local write "Retract Pump 1"(FALSE ("Retract Pump 1")) -> ()
        n1591 = case shown="True" "Retract Pump 1" {
          tunnel: w2259 -> [_ w2264]
          frame False {
          }
          frame True {
            n1592 = local read "Retract Rate (mL/m)"() -> (w2262:dbl)
            n1593 = Number To Decimal String(number=w2262) -> (decimal integer string=w2280:string)  [unwired: 1 in]
            n1594 = Concatenate Strings("wrate  " ("string"), w2280, " u/m" ("string"), "\r") -> (w2282:string)
            n1595 = VISA Write(VISA resource name=w2264, write buffer=w2282) -> (VISA resource name out=w2274:refnum<visa-resource-name>)  [unwired: 1 in, 2 out]
            n1596 = Number To Decimal String(number="Retract Vol 1 (uL)") -> (decimal integer string=w2276:string)  [unwired: 1 in]
            n1597 = Concatenate Strings("tvolume  " ("string"), w2276, " u" ("string"), "\r") -> (w2273:string)
            n1598 = VISA Write(VISA resource name=w2274, write buffer=w2273) -> (VISA resource name out=w2270:refnum<visa-resource-name>)  [unwired: 1 in, 2 out]
            n1599 = Concatenate Strings("cvolume" ("string"), "\r") -> (w2271:string)
            n1600 = VISA Write(VISA resource name=w2270, write buffer=w2271) -> (VISA resource name out=w2265:refnum<visa-resource-name>)  [unwired: 1 in, 2 out]
            n1601 = Concatenate Strings("wrun" ("string"), "\r") -> (w2266:string)
            n1602 = VISA Write(VISA resource name=w2265, write buffer=w2266) -> ()  [unwired: 1 in, 3 out]
          }
        }
      }
      event "Flip Green Filter": Value Change {
        n1603 = event-data() -> ()  [unwired: 7 out]
        n1604 = Not(x="Flip Green Filter") -> (.not. x?=w2284:bool)
        n1605 = local write "Flip Green Filter"(w2284) -> ()
        n1606 = flat-sequence {
          tunnel: w2292 -> [w2297]
          tunnel: w2291 -> [w2296]
          tunnel: [w2294] -> w2289
          tunnel: [w2293] -> w2288
          tunnel: [w2299] -> w2287
          tunnel: w2289 -> [w2299]
          tunnel: [w2298] -> w2286
          tunnel: w2288 -> [w2298]
          tunnel: w2287 -> [w2303]
          tunnel: w2286 -> [w2302]
          tunnel: [w2301] -> w2290
          frame #0 {
            n1607 = xnode "Read/Write Control"("FPGA VI Reference In"=w2297, "error in"=w2296, "Green Filter Flipper"=TRUE) -> ("FPGA VI Reference Out"=w2294:T22, "error out"=w2293:errorcluster)
          }
          frame #1 {
            n1608 = Wait (ms)(milliseconds to wait=u32 100) -> ()  [unwired: 1 out]
          }
          frame #2 {
            n1609 = xnode "Read/Write Control"("FPGA VI Reference In"=w2303, "error in"=w2302, "Green Filter Flipper"=FALSE) -> ("error out"=w2301:errorcluster)  [unwired: 1 out]
          }
        }
      }
      event "Pump 1 contents", "Pump 3 contents": Value Change {
        n1610 = event-data() -> ()  [unwired: 7 out]
        n1611 = local read "Pump 1 contents"() -> (→"Pump 1 cont disp":string)
        n1612 = local read "Pump 3 contents"() -> (→"Pump 3 cont disp":string)
      }
      event "Reset Trap Pos. FB": Value Change {
        n1613 = event-data() -> ()  [unwired: 7 out]
        n1614 = xnode "Read/Write Control"("FPGA VI Reference In"=w2309, "error in"=w2308, "Trap Pos. FB Reset"="Reset Trap Pos. FB") -> ()  [unwired: 2 out]
      }
      event "Rem fb disp offset": Value Change {
        n1615 = event-data() -> ()  [unwired: 7 out]
        n1616 = local write "Rem fb disp offset"(FALSE ("Rem fb disp offset")) -> ()
        n1617 = local read "Mean T1 Position (nm)"() -> (w2311:dbl)
        n1618 = local read "FB Trap Pos Offset"() -> (w2312:dbl)
        n1619 = Subtract(x=w2312, y=w2311) -> (x-y=w2310:dbl)
        n1620 = local write "FB Trap Pos Offset"(w2310) -> ()
      }
      event "Threshold (nm)": Value Change {
        n1621 = event-data() -> ()  [unwired: 7 out]
        n1622 = flat-sequence {
          tunnel: w2316 -> [w2324]
          tunnel: w2315 -> [w2323]
          tunnel: [w2317] -> w2314
          tunnel: w2314 -> [w2330]
          frame #0 {
            n1623 = xnode "Read/Write Control"("FPGA VI Reference In"=w2324, "error in"=w2323) -> ("FPGA VI Reference Out"=w2320:T22, "error out"=w2319:errorcluster, "FPGA TTrig Thresh"=w2321:i64)
            n1624 = local read "Threshold stored (nm)"() -> (w2329:dbl)
            n1625 = local read "Threshold (nm)"() -> (w2317:dbl)
            n1626 = local read "AOM X Cal (nm/MHz)"() -> (w2327:dbl)
            n1627 = Subtract(x=w2317, y=w2329) -> (x-y=w2328:dbl)
            n1628 = Divide(x=w2328, y=w2327) -> (x/y=w2325:dbl)
            n1629 = call "IR AOM freq to word.vi"("Frequency In (MHz)"=w2325) -> ("Frequency Word Out (double)"=w2326:dbl)
            n1630 = To Quad Integer(1:w2326) -> (0:w2322:i64)
            n1631 = Add(x=w2321, y=w2322) -> (x+y=w2318:i64)
            n1632 = xnode "Read/Write Control"("FPGA VI Reference In"=w2320, "error in"=w2319, "FPGA TTrig Thresh"=w2318) -> ()  [unwired: 2 out]
          }
          frame #1 {
            "Threshold stored (nm)" <- w2330
          }
        }
      }
      event "FB Trig Integrate": Value Change {
        n1633 = event-data() -> ()  [unwired: 7 out]
        n1634 = local read "FB Trig Integrate"() -> (w2332:u32)
        n1635 = xnode "Read/Write Control"("FPGA VI Reference In"=w2334, "error in"=w2333, "FB Trig Integrate"=w2332) -> ("error out"=w2331:errorcluster)  [unwired: 1 out]
      }
      event "11": Value Change {
        n1636 = event-data() -> ()  [unwired: 7 out]
        n1637 = local read "11"() -> (w2335:bool)
        n1638 = case shown="True" w2335 {
          frame False {
          }
          frame True {
            n1639 = local read "Messages"() -> (w2337:string)
            n1640 = call "Update messages.vi"("Message to add"="You kicked it up to 11!", "Old message string"=w2337) -> ("New message string"=w2338:string)
            n1641 = call <vilib>:"Beep.vi"() -> ()  [unwired: 12 in]
            n1642 = local write "Messages"(w2338) -> ()
          }
        }
      }
      event "Trap Pos. FB ON": Value Change {
        n1643 = event-data() -> ()  [unwired: 7 out]
        n1644 = xnode "Read/Write Control"("FPGA VI Reference In"=w2341, "error in"=w2340, "Force feedback"="Trap Pos. FB ON") -> ()  [unwired: 2 out]
      }
      event "Remove Action Offset": Value Change {
        n1645 = event-data() -> ()  [unwired: 7 out]
        n1646 = local write "Remove Action Offset"(FALSE ("Remove Action Offset")) -> ()
        n1647 = local read "Trap Pos. FB Mult Factor"() -> (w2346:i64)
        n1648 = local read "Trap Pos FB Action"() -> (w2344:i64)
        n1649 = local read "Trap Pos. FB Offset Factor"() -> (w2342:i64)
        n1650 = Multiply(x=w2346, y=w2344) -> (x*y=w2345:i64)
        n1651 = Add(x=w2345, y=w2342) -> (x+y=w2343:i64)
        n1652 = local write "Trap Pos. FB Offset Factor"(w2343) -> ()
        n1653 = xnode "Read/Write Control"("FPGA VI Reference In"=w2349, "error in"=w2348, "Trap Pos. FB Offset Factor"=w2343) -> ()  [unwired: 2 out]
      }
      event "Remove Offset to factor": Value Change {
        n1654 = event-data() -> ()  [unwired: 7 out]
        n1655 = local write "Remove Offset to factor"(FALSE ("Remove Action Offset")) -> ()
        n1656 = local read "Trap Pos. FB Mult Factor"() -> (w2361:i64)
        n1657 = local read "Trap Pos FB Action"() -> (w2359:i64)
        n1658 = local read "Trap Pos. FB Offset Factor"() -> (w2358:i64)
        n1659 = Multiply(x=w2361, y=w2359) -> (x*y=w2360:i64)
        n1660 = local read "Trap Pos. FB Mult Factor"() -> (w2357:i64)
        n1661 = Add(x=w2360, y=w2358) -> (x+y=w2352:i64)
        n1662 = Multiply(x=32768, y="factor") -> (x*y=w2355:dbl)
        n1663 = Multiply(x=w2355, y=w2357) -> (x*y=w2356:dbl)
        n1664 = Subtract(x=w2352, y=w2356) -> (x-y=w2350:dbl)
        n1665 = To Quad Integer(1:w2350) -> (0:w2351:i64)
        n1666 = xnode "Read/Write Control"("FPGA VI Reference In"=w2364, "error in"=w2363, "Trap Pos. FB Offset Factor"=w2351) -> ()  [unwired: 2 out]
        n1667 = local write "Trap Pos. FB Offset Factor"(w2351) -> ()
      }
      event "Trap Pos. FB Range", "Trap Pos. FB Gains", "Trap Pos. FB Mult Factor", "Trap Pos. FB Offset Factor", "Trap Pos FB Negate Action", "Trap Pos FB Monitor\nT1 or T2", "Differential FB?", "Negate Diff?": Value Change {
        n1668 = event-data() -> ()  [unwired: 7 out]
        n1669 = local read "Negate Diff?"() -> (w2365:bool)
        n1670 = xnode "Read/Write Control"("FPGA VI Reference In"=w2375, "error in"=w2374, "Trap Pos. FB Range"="Trap Pos. FB Range", "Trap Pos. FB Gains"="Trap Pos. FB Gains", "Trap Pos. FB Mult Factor"="Trap Pos. FB Mult Factor", "Trap Pos. FB Offset Factor"="Trap Pos. FB Offset Factor", "Trap Pos FB Negate Action"="Trap Pos FB Negate Action", "Trap Pos FB Monitor T1 or T2"="Trap Pos FB Monitor\nT1 or T2", "AI1 X Scale"="Trap Pos. AI1 X Pre-scale", "Negate Diff?"=w2365, "Diff FB Measurement?"="Differential FB?") -> ()  [unwired: 2 out]
      }
      event "Trap Pos FB SP", "Trap Pos FB SP 2", "Use SP 2": Value Change {
        n1671 = event-data() -> ()  [unwired: 7 out]
        n1672 = Select(t="Trap Pos FB SP 2", s="Use SP 2", f="Trap Pos FB SP") -> (s? t:f=w2376:fxp<+/-,16,1>)
        n1673 = xnode "Read/Write Control"("FPGA VI Reference In"=w2381, "error in"=w2380, "Trap Pos. FB SP"=w2376) -> ()  [unwired: 2 out]
      }
      event "Offset SP2 from SP1": Value Change {
        n1674 = event-data() -> ()  [unwired: 7 out]
        n1675 = local read "Trap Pos FB SP"() -> (w2384:fxp<+/-,16,1>)
        n1676 = Add(x=w2384, y="SP2 Offset") -> (x+y=w2382:fxp<+/-,16,1>)
        n1677 = property on="Trap Pos FB SP 2" class="DigNum (strict)"("Val(Sgnl)"=w2382) -> ()  [unwired: 2 in, 2 out]
        n1678 = local write "Offset SP2 from SP1"(FALSE ("Offset SP2 from SP1")) -> ()
      }
      event "Set Reading to\nSetpoint": Value Change {
        # "This is the actual PID input signal"
        n1679 = event-data() -> ()  [unwired: 7 out]
        n1680 = local write "Set Reading to\nSetpoint"(FALSE ("Set SP to Reading")) -> ()
        n1681 = xnode "Read/Write Control"("FPGA VI Reference In"=w2390, "error in"=w2389) -> ("FPGA VI Reference Out"=w2388:T22, "error out"=w2387:errorcluster, "Trap Pos FB Int-Norm Signal"=w2386:fxp<+/-,16,1>)
        n1682 = local read "Differential FB?"() -> (w2391:bool)
        n1683 = case shown="False" w2391 {
          tunnel: [w2396 w2403] -> w2393
          tunnel: w2386 -> [w2394 w2403]
          frame False {
            n1684 = local read "Trap Pos FB Monitor\nT1 or T2"() -> (w2399:bool)
            n1685 = local read "Trap X AI1 (DMA)"() -> (w2402:T13)
            n1686 = Unbundle By Name(w2402) -> ("Set 1"=w2401:fxp<+/-,16,1>, "Set 2"=w2400:fxp<+/-,16,1>)
            n1687 = Select(t=w2401, s=w2399, f=w2400) -> (s? t:f=w2398:fxp<+/-,16,1>)
            n1688 = Not(x="Set SP Using...") -> (.not. x?=w2395:bool)
            n1689 = Select(t=w2394, s=w2395, f=w2398) -> (s? t:f=w2396:fxp<+/-,16,1>)
          }
          frame True {
          }
        }
        n1690 = xnode "Read/Write Control"("FPGA VI Reference In"=w2388, "error in"=w2387, "Trap Pos. FB SP"=w2393) -> ()  [unwired: 2 out]
        n1691 = local write "Trap Pos FB SP"(w2393) -> ()
      }
      event "Trap Pos. FB Out Scale 2^n": Value Change {
        n1692 = event-data() -> ()  [unwired: 7 out]
        n1693 = Scale By Power Of 2(n="Trap Pos. FB Out Scale 2^n", x=ext 1.0) -> (x*2^n=w2404:ext)
        n1694 = property on="Trap Pos. FB Mult Factor" class="DigNum (strict)"("Val(Sgnl)"=w2404) -> ()  [unwired: 2 in, 2 out]
      }
      event "Trap Pos FB Int Count": Value Change {
        n1695 = event-data() -> ()  [unwired: 7 out]
        n1696 = xnode "Read/Write Control"("FPGA VI Reference In"=w2409, "error in"=w2408, "Trap Pos FB Int Count"="Trap Pos FB Int Count") -> ()  [unwired: 2 out]
      }
      event "Trap pos": Value Change {
        n1697 = event-data() -> ()  [unwired: 7 out]
        n1698 = case shown="True" "Trap pos" {
          frame False {
            n1699 = property on="Trap Delta Graph" class="WFGraph (strict)"("Visible"=TRUE) -> ()  [unwired: 2 in, 2 out]
            n1700 = property on="Saved trap pos" class="WFGraph (strict)"("Visible"=FALSE) -> ()  [unwired: 2 in, 2 out]
          }
          frame True {
            n1701 = property on="Saved trap pos" class="WFGraph (strict)"("Visible"=TRUE) -> ()  [unwired: 2 in, 2 out]
            n1702 = property on="Trap Delta Graph" class="WFGraph (strict)"("Visible"=FALSE) -> ()  [unwired: 2 in, 2 out]
          }
        }
      }
      event "Save user params": Value Change {
        n1703 = event-data() -> ()  [unwired: 7 out]
        n1704 = local write "Save user params"(FALSE ("Save user\nparams")) -> ()
        n1705 = call "save control values.vi"("User"="User") -> ()  [unwired: 8 in, 1 out]
        n1706 = local read "Messages"() -> (w2421:string)